vi "Laser Ablation and Capture.vi"() -> ()   [LabVIEW 2016]
uses:
  System.Windows.Forms
  D:/Fabrizio/Labview Projects/VersionControlled/Laser Ablation Capture Software/uc480DotNet.dll
  uc480DotNet.dll
  <vilib>/Utility/miscctls.llb/LVBoundsTypeDef.ctl
  <vilib>/regexp/Match Regular Expression.xnode
  <vilib>/vision/NI_Vision_Development_Module.lvlib
  <vilib>/Utility/config.llb/NI_LVConfig.lvlib
panel:
  in  "Load ROI":bool
  in  "Save current ROI":bool
  in  "Call Last ROI":bool
  in  "Captur time\nConstant":dbl=0.001 min=0.001 step=0.001 format="%#_13g"
  out "Pre-Capture Axis 2":dbl format="%.10e"
  out "Pre-Capture Axis 1":dbl format="%.10e"
  in  "Log files":bool
  out "Axis 2 inverted?":bool
  out "Axis 1 inverted?":bool
  out "Rect height\n(px)":i32
  out "Rect width\n(px)":i32
  in  "Circle?":bool=TRUE
  out "Axis 2 group":i32
  out "Axis 1 group":i32
  in  "Microscope/Capture \nstatus button":bool=TRUE
  in  "X travel":dbl min=0.0 max=150.0 step=0.0001
  in  "Y travel":dbl min=0.0 max=150.0 step=0.0001
  in  "Laser Status":bool
  in  "SINGLE SHOT":bool
  in  "Repetition\nRate (Hz)":dbl=2.34 min=1.0 max=20.0 step=0.01 format="%.2g"
  out "Laser Com Delay":i32
  out "VISA Laser port":string
  in  "Acceleration \n(mm/s²)":dbl=20.0
  out "Camera Status":string="Load parameter"
  in  "Save configuration":bool
  in  "Stages status":bool
  in  "Transparency":u8 max=80 step=1
  in  "Overlay MSI Image":bool
  in  "Home Axes":bool
  out "Axis 2 Offset":dbl
  out "Axis 1 Offset":dbl
  out "Acceleration":dbl
  out "Velocity":dbl
  in  "Axis Initial Parameters":T1={"Velocity (units/seconds)"=1.0, "Acceleration (units/seconds²)"=20.0, "Minimum Jerk Time (seconds)"=0.005, "Maximum Jerk Time (seconds)"=0.009} {"Maximum Jerk Time (seconds)" format="%.6e"; "Minimum Jerk Time (seconds)" format="%.6e"; "Acceleration (units/seconds²)" format="%.6e"; "Velocity (units/seconds)" format="%.6e"}
  out "Axis 2":string
  out "Axis 1":string
  out "XPS_Address":string
  in  "Axes Manual Control":bool
  out "ROI Area \n(mm2)":dbl=4.035870075999999
  out "Laser on/off array":bool[][](array[boolean])
  out "Commands array":string[][](array[string])
  in  "Exit Camera":bool
  in  "Width (px)":i32=240
  in  "X offset":i32=406 step=1
  in  "Y offset":i32=693 step=1
  out "Processi time (sec)":i32=117
  in  "Processing time unit":string(combo)="sec"
  out "Process time":dbl=117.0
  in  "Mode":i32(ring) items=["RGB 32"=0, "RGB 24"=1, "Y8 Monochrom"=6]
  in  "Camera":refnum<k24>(container)
  in  "Init Camera":bool
  in  "Start Live":bool
  in  "Stop Live":bool
  in  "Load Parameter":bool
  out "Error Out":errorcluster caption="error"
  out "Bits/Pixel":i32=32
  out "Width":i32=1280
  out "Height":i32=1024
  out "Serial Number":string="4102944807"
  in  "Camera ID":i32
  in  "Zoom":dbl(ring)=1.5 items=["4X"=4.0, "2X"=2.0, "1.5X"=1.5, "1.25X"=1.25, "1X"=1.0]
  in  "Gain Boost":bool=TRUE
  in  "Snapshot":bool
  out "Output":picture
  in  "Exposure":dbl(slide)=99.80425000000001 min=0.06241666666666667 max=99.80425000000001 step=0.06241666666666667 scale=0.06241666666666667..99.80425000000001 scale format="%#.3g"
  in  "Framerate":dbl(slide)=10.002522802986672 min=0.47411700449083627 max=15.001275108384213 step=0.014032998230481021 scale=0.47411700449083627..15.001275108384213 scale format="%#.3g"
  in  "Pixelclock":i32(slide)=24 min=5 max=40 step=1 scale=5.0..40.0
  in  "error in (no error)":errorcluster
  out "error out":errorcluster
  in  "Precision (%)":dbl=1.0 min=1.0 max=100.0 step=1.0 format="%#_3g"
  in  "Process Image":bool
  in  "Pixel size":dbl=12.19 step=0.01
  in  "Speed (µm/s)":i32=1000
  in  "Heigth (px)":i32=240
  in  "Height \nstep divider":i32=2
  out "Rect height\n(µm/px)":i32=2267
  out "Rect. width \n(µm/px))":i32=2267
  out "Source":T2(plugin-control)
  in  "Open \nManual":bool
  in  "Capture":bool
  out "Log":string
  out "Laser Operation":bool
  in  "LASER":bool
  in  "LAMP":bool
  in  "EXIT":bool
  # "Laser Control"
  # "Stages Control"
  # "Camera Control"
  # "ROI Processing"
  # "Laser spot size and position"
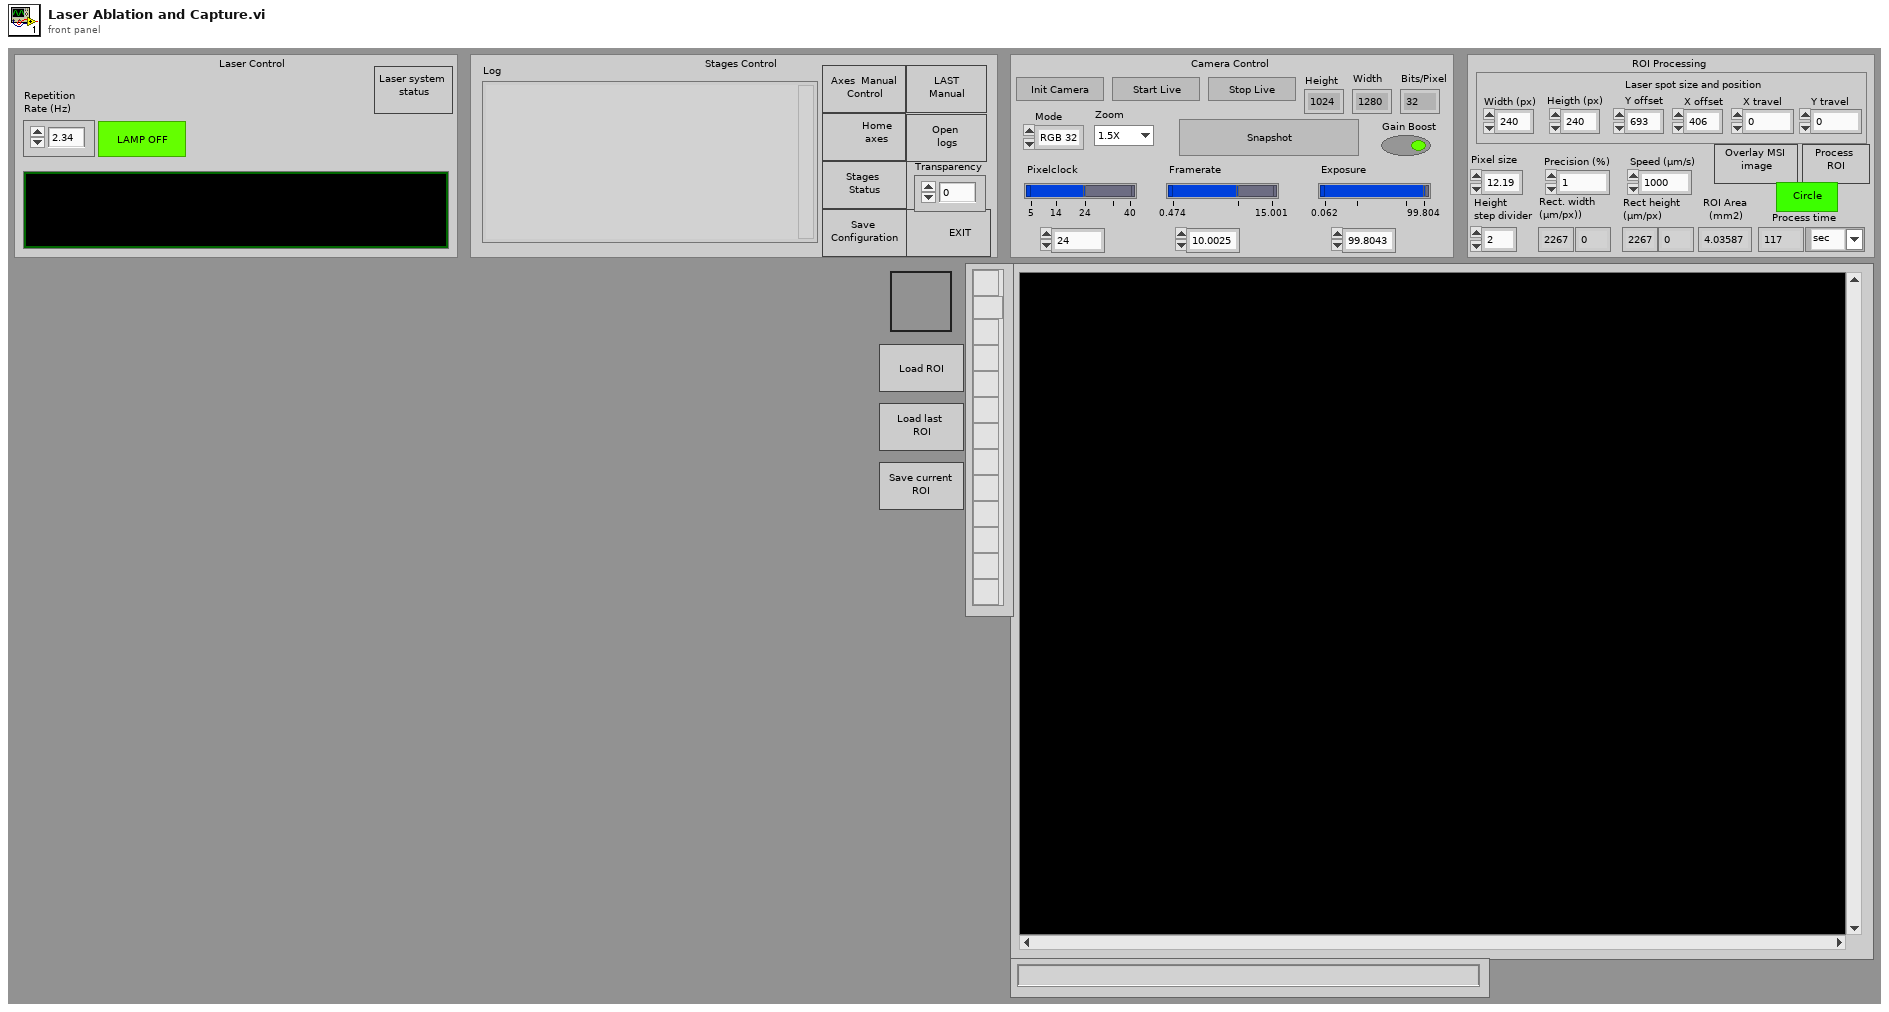
[diagram p1: front panel]
types:
  T1 = cluster{"Velocity (units/seconds)":dbl, "Acceleration (units/seconds²)":dbl, "Minimum Jerk Time (seconds)":dbl, "Maximum Jerk Time (seconds)":dbl}
  T2 = typedef "IMAQ Image.ctl" = refnum<image>
  T3 = typedef "LVBoundsTypeDef.ctl" = cluster{"Width":u32, "Height":u32}
  T4 = enum8{"Enabled", "Disabled", "Disabled and Grayed Out"}
  T5 = typedef "NI_LVConfig.lvlib/Config Data RefNum.ctl" = refnum<k1>
  T6 = enum16{"open", "replace", "create", "open or create", "replace or create", "replace or create with confirmation"}
  T7 = enum32{"Invalid", "Standard", "Closed", "Hidden", "Minimized", "Maximized"}
  T8 = enum32{"invalid app kind", "Development System", "Run Time System", "Student Edition", "Embedded LabVIEW", "Evaluation", "Custom"}
  T9 = cluster{"connection TCP":refnum<k5>, "LogTo File":bool, "Log File refnum":refnum<file>, "no error if error log":bool}
  T10 = cluster{"Global Rectangle":i32[], "Contours":cluster{"Contour Type":u32, "ROI Type":u32, "Points":i32[]}[]}
  T11 = typedef "ROI Descriptor" = cluster{"Global Rectangle":i32[], "Contours":cluster{"ID":enum32{"External", "Internal"}, "Type":u32, "Coordinates":i32[]}[]}
  T12 = cluster{"ID":enum32{"External", "Internal"}, "Type":u32, "Coordinates":i32[]}[]
  T13 = cluster{"ID":enum32{"External", "Internal"}, "Type":u32, "Coordinates":i32[]}
  T14 = cluster{"Contour Type":u32, "ROI Type":u32, "Points":i32[]}[]
  T15 = cluster{"Contour Type":u32, "ROI Type":u32, "Points":i32[]}
diagram:
  w63 = 682  # Height
  w64 = 853  # Width
  w65 = 1 items=["None", "FixedSingle", "Fixed3D"]  # BorderStyle
  w69 = u8 2  # Deaktiviert
  w70 = u8 2  # Deaktiviert
  w72 = u8 2  # Deaktiviert
  w73 = u8 0  # Deaktiviert
  # "Button and controls"
  # "Camera control buttons"
  n1 = property on="Property Node" class="PictureBox"(reference="Camera", "BorderStyle"=w65, "Width"=w64, "Height"=w63) -> (reference out=w53:refnum<k24>, error out=w54:errorcluster)  [unwired: 1 in]
  n2 = property on="Property Node" class="PictureBox"(reference=w53, error in=w54) -> (reference out=w52:refnum<k24>, error out=w51:errorcluster, "Handle"=w50:refnum<k24>)
  n3 = while "Camera Control" {
    shift-right: [w82] -> _
    shift-left: w51 -> [w88]
    shift-right: [w85] -> _
    shift-left: _ -> [w78]
    shift-right: [w80] -> _
    shift-left: w52 -> [w81]
    tunnel: w50 -> [w79]
    stop <- w86 stop-if-true
    # ".NetReference"
    # ".Net Reference"
    n4 = event shown="[1] Timeout" {
      selector: _ -> [_ _]
      dyn-events: _ -> [_ _]
      timeout: 0 -> [_ _]
      event "Load Parameter", "Start Live": Mouse Down {
        n5 = event-data() -> ()  [unwired: 1 in, 2 out]
      }
      event Timeout {
        n6 = event-data() -> ()  [unwired: 1 in, 2 out]
      }
    }
    n7 = event shown="[1] Timeout" {
      selector: _ -> [_ _]
      dyn-events: _ -> [_ _]
      timeout: 0 -> [_ _]
      tunnel: [w102 w113] -> w89
      tunnel: w88 -> [w112 w113]
      tunnel: w78 -> [w111 _]
      event "Pixelclock": Value Change; "Pixelclock": Mouse Move; "Pixelclock": Key Down; "Pixelclock": Mouse Up {
        n8 = event-data() -> ("CtlRef"=w104:refnum<vi>)  [unwired: 1 in, 3 out]
        n9 = call "uc480_SubVI_Example_GetFramerate.vi"(".NET (Reference)"=w111, "Error In"=w112) -> ("Framerate"=w110:dbl, "Inc"=w109:dbl, "Min"=w107:dbl, "Max"=w108:dbl, "error out"=w106:errorcluster)  [unwired: 9 in]
        n10 = property on="Framerate" class="Slide (strict)"(error in=w106, "Value"=w110, "Increment"=w109, "Minimum"=w107, "Maximum"=w108) -> (error out=w105:errorcluster)  [unwired: 1 in, 1 out]
        n11 = property on="Framerate" class="Slide (strict)"(error in=w105, "Scale.Increment"=w109, "Scale.Minimum"=w107, "Scale.Maximum"=w108) -> (error out=w103:errorcluster)  [unwired: 1 in, 1 out]
        n12 = Close Reference(reference=w104, error in (no error)=w103) -> (error out=w102:errorcluster)
      }
      event Timeout {
        n13 = event-data() -> ()  [unwired: 1 in, 2 out]
      }
    }
    n14 = case shown="False" "Load Parameter" {
      tunnel: ["" "Load parameter"] -> w95
      frame False {
      }
      frame True {
      }
    }
    n15 = case shown="False" "Init Camera" {
      tunnel: ["" "Init camera"] -> w99
      frame False {
      }
      frame True {
      }
    }
    n16 = case shown="False" "Exit Camera" {
      tunnel: ["" "Exit camera"] -> w93
      frame False {
      }
      frame True {
      }
    }
    n17 = event shown="[1] Timeout" {
      selector: _ -> [_ _]
      dyn-events: _ -> [_ _]
      timeout: 0 -> [_ _]
      tunnel: w89 -> [w124 w125]
      tunnel: [w114 w125] -> w91
      tunnel: w78 -> [w123 _]
      event "Pixelclock", "Framerate": Value Change; "Pixelclock", "Framerate": Mouse Move; "Pixelclock", "Framerate": Key Down; "Pixelclock", "Framerate": Mouse Up {
        n18 = event-data() -> ("CtlRef"=w116:refnum<vi>)  [unwired: 1 in, 3 out]
        n19 = call "uc480_SubVI_Example_GetExposure.vi"(".NET (Reference)"=w123, "Error In"=w124) -> ("Exposure"=w120:dbl, "Inc"=w119:dbl, "Min"=w118:dbl, "Max"=w117:dbl, "Error out"=w121:errorcluster)  [unwired: 9 in]
        n20 = property on="Exposure" class="Slide (strict)"(error in=w121, "Value"=w120, "Increment"=w119, "Minimum"=w118, "Maximum"=w117) -> (error out=w122:errorcluster)  [unwired: 1 in, 1 out]
        n21 = property on="Exposure" class="Slide (strict)"(error in=w122, "Scale.Increment"=w119, "Scale.Minimum"=w118, "Scale.Maximum"=w117) -> (error out=w115:errorcluster)  [unwired: 1 in, 1 out]
        n22 = Close Reference(reference=w116, error in (no error)=w115) -> (error out=w114:errorcluster)
      }
      event Timeout {
        n23 = event-data() -> ()  [unwired: 1 in, 2 out]
      }
    }
    n24 = case shown="False" "Start Live" {
      tunnel: ["" "Start live"] -> w98
      frame False {
      }
      frame True {
      }
    }
    n25 = case shown="False" "Stop Live" {
      tunnel: ["" "Stop live"] -> w94
      frame False {
      }
      frame True {
      }
    }
    n26 = local read "Camera Status"() -> (w75:string)
    n27 = Concatenate Strings(w99, w98, w95, w94, w93) -> (→"Camera Status":string)
    n28 = case shown="Default" w75 {
      tunnel: w78 -> [w168 w208 w266 w308 w488 w547]
      tunnel: w91 -> [w171 w209 w267 w318 w487 w548]
      tunnel: [w142 w207 w275 w317 w446 w546] -> w85
      tunnel: [w143 w206 w276 w316 w483 w544] -> w84
      tunnel: [FALSE FALSE TRUE FALSE FALSE FALSE] -> w86
      tunnel: w81 -> [w141 w200 w248 w300 w441 w537]
      tunnel: [w141 w200 w247 w299 w441 w537] -> w80
      tunnel: w79 -> [_ _ _ w296 _ _]
      frame "Load parameter" {
        # "SubVI Example for \nMemory allocation"
        # "Is acquisition running?"
        # "Load Parameter"
        n29 = property class="Camera"(reference=w168, error in=w171) -> (error out=w176:errorcluster, "Acquisition"=w175:refnum<k24>)  [unwired: 1 out]
        n30 = invoke class="Acquisition" method="HasStarted"(reference=w175, error in=w176) -> (reference out=w172:refnum<k24>, error out=w174:errorcluster, "bValue"=w170:bool)  [unwired: 2 in, 1 out]
        n31 = control-ref of="Start Live"() -> (w166:refnum<vi>)
        n32 = invoke class="Acquisition" method="ToString"(reference=w172, error in=w174) -> (reference out=w138:refnum<k24>, error out=w137:errorcluster, "ToString"=w173:string)  [unwired: 1 in]
        n33 = property class="Bool"(reference=w166, "Disabled"=u8 0 ("Deaktiviert")) -> (reference out=w140:refnum<vi>, error out=w139:errorcluster)  [unwired: 1 in]
        n34 = Close Reference(reference=w138, error in (no error)=w137) -> (error out=w136:errorcluster)
        n35 = Close Reference(reference=w140, error in (no error)=w139) -> ()  [unwired: 1 out]
        n36 = call "uc480_Error_Handling.vi"("Error String"=w173, "Error In"=w136) -> ("Error Out"=w169:errorcluster)  [unwired: 9 in]
        n37 = case shown="False" w170 {
          tunnel: w169 -> [w184 w191]
          tunnel: w168 -> [w182 w192]
          tunnel: [w183 w191] -> w167
          tunnel: [w182 w192] -> w142
          frame False {
            n38 = property class="Camera"(reference=w182, error in=w184) -> (error out=w186:errorcluster, "Parameter"=w185:refnum<k24>)  [unwired: 1 out]
            n39 = invoke class="Parameter" method="Load"(reference=w185, error in=w186, "strFilename"="") -> (reference out=w188:refnum<k24>, error out=w189:errorcluster, "Load"=w181:i32)  [unwired: 1 in, 1 out]
            n40 = invoke class="Parameter" method="ToString"(reference=w188, error in=w189) -> (reference out=w178:refnum<k24>, error out=w180:errorcluster, "ToString"=w190:string)  [unwired: 1 in]
            n41 = Close Reference(reference=w178, error in (no error)=w180) -> (error out=w179:errorcluster)
            n42 = call "uc480_Error_Handling.vi"("Error Code"=w181, "Error String"=w190, "Error In"=w179) -> ("Error Out"=w183:errorcluster)  [unwired: 8 in]
          }
          frame True {
          }
        }
        n43 = call "uc480_SubVI_Example_MemoryAllocation.vi"(".NET (Reference)"=w142, "Error In"=w167) -> ("Error Out"=w144:errorcluster)  [unwired: 13 in, 4 out]
        n44 = call "uc480_SubVI_Example_GetPixelClock.vi"(".NET (Reference)"=w142, "Error In"=w144) -> ("Pixel Clock"=w145:i32, "Inc"=w147:i32, "Min"=w148:i32, "Max"=w149:i32, "error out"=w146:errorcluster)  [unwired: 9 in]
        n45 = property on="Pixelclock" class="Slide (strict)"(error in=w146, "Value"=w145, "Increment"=w147, "Minimum"=w148, "Maximum"=w149) -> (error out=w150:errorcluster)  [unwired: 1 in, 1 out]
        n46 = property on="Pixelclock" class="Slide (strict)"(error in=w150, "Scale.Increment"=w147, "Scale.Minimum"=w148, "Scale.Maximum"=w149) -> (error out=w151:errorcluster)  [unwired: 1 in, 1 out]
        n47 = call "uc480_SubVI_Example_GetFramerate.vi"(".NET (Reference)"=w142, "Error In"=w151) -> ("Framerate"=w154:dbl, "Inc"=w155:dbl, "Min"=w156:dbl, "Max"=w157:dbl, "error out"=w153:errorcluster)  [unwired: 9 in]
        n48 = property on="Framerate" class="Slide (strict)"(error in=w153, "Value"=w154, "Increment"=w155, "Minimum"=w156, "Maximum"=w157) -> (error out=w152:errorcluster)  [unwired: 1 in, 1 out]
        n49 = property on="Framerate" class="Slide (strict)"(error in=w152, "Scale.Increment"=w155, "Scale.Minimum"=w156, "Scale.Maximum"=w157) -> (error out=w158:errorcluster)  [unwired: 1 in, 1 out]
        n50 = call "uc480_SubVI_Example_GetExposure.vi"(".NET (Reference)"=w142, "Error In"=w158) -> ("Exposure"=w161:dbl, "Inc"=w162:dbl, "Min"=w163:dbl, "Max"=w164:dbl, "Error out"=w159:errorcluster)  [unwired: 9 in]
        n51 = property on="Exposure" class="Slide (strict)"(error in=w159, "Value"=w161, "Increment"=w162, "Minimum"=w163, "Maximum"=w164) -> (error out=w160:errorcluster)  [unwired: 1 in, 1 out]
        n52 = property on="Exposure" class="Slide (strict)"(error in=w160, "Scale.Increment"=w162, "Scale.Minimum"=w163, "Scale.Maximum"=w164) -> (error out=w143:errorcluster)  [unwired: 1 in, 1 out]
      }
      frame "Stop live" {
        # "Is acquisition running?"
        # "Stop Acquisition"
        n53 = property class="Camera"(reference=w208, error in=w209) -> (error out=w216:errorcluster, "Acquisition"=w215:refnum<k24>)  [unwired: 1 out]
        n54 = invoke class="Acquisition" method="HasStarted"(reference=w215, error in=w216) -> (reference out=w210:refnum<k24>, error out=w212:errorcluster, "bValue"=w214:bool)  [unwired: 2 in, 1 out]
        n55 = control-ref of="Load Parameter"() -> (w204:refnum<vi>)
        n56 = control-ref of="Start Live"() -> (w201:refnum<vi>)
        n57 = invoke class="Acquisition" method="ToString"(reference=w210, error in=w212) -> (reference out=w193:refnum<k24>, error out=w195:errorcluster, "ToString"=w211:string)  [unwired: 1 in]
        n58 = property class="Bool"(reference=w204, "Disabled"=u8 0 ("Deaktiviert")) -> (reference out=w199:refnum<vi>, error out=w198:errorcluster)  [unwired: 1 in]
        n59 = property class="Bool"(reference=w201, "Disabled"=u8 0 ("Deaktiviert")) -> (reference out=w197:refnum<vi>, error out=w196:errorcluster)  [unwired: 1 in]
        n60 = Close Reference(reference=w193, error in (no error)=w195) -> (error out=w194:errorcluster)
        n61 = Close Reference(reference=w199, error in (no error)=w198) -> ()  [unwired: 1 out]
        n62 = Close Reference(reference=w197, error in (no error)=w196) -> ()  [unwired: 1 out]
        n63 = call "uc480_Error_Handling.vi"("Error String"=w211, "Error In"=w194) -> ("Error Out"=w213:errorcluster)  [unwired: 9 in]
        n64 = case shown="True" w214 {
          tunnel: [w218 w237] -> w206
          tunnel: w213 -> [w218 w238]
          tunnel: w208 -> [w217 w230]
          tunnel: [w217 w230] -> w207
          frame False {
          }
          frame True {
            n65 = property class="Camera"(reference=w230, error in=w238) -> (error out=w234:errorcluster, "Acquisition"=w235:refnum<k24>)  [unwired: 1 out]
            n66 = invoke class="Acquisition" method="Stop"(reference=w235, error in=w234) -> (reference out=w232:refnum<k24>, error out=w233:errorcluster, "Stop"=w231:i32)  [unwired: 1 in]
            n67 = invoke class="Acquisition" method="ToString"(reference=w232, error in=w233) -> (reference out=w227:refnum<k24>, error out=w229:errorcluster, "ToString"=w236:string)  [unwired: 1 in]
            n68 = Close Reference(reference=w227, error in (no error)=w229) -> (error out=w228:errorcluster)
            n69 = call "uc480_Error_Handling.vi"("Error Code"=w231, "Error String"=w236, "Error In"=w228) -> ("Error Out"=w237:errorcluster)  [unwired: 8 in]
            n70 = Get Date/Time In Seconds() -> (seconds since 1Jan1904=w225:timestamp)
            n71 = Format Date/Time String(time format string (%c)="%m/%d/%y - %I:%M %p  ", seconds (now)=w225) -> (date/time string=w226:string)  [unwired: 1 in]
            n72 = Concatenate Strings(w226, "Camera stopped", "\r") -> (w221:string)
            n73 = invoke on="Log" class="Str" method="Append String"("string"=w221) -> (error out=w219:errorcluster)  [unwired: 3 in, 3 out]
            n74 = property on="Log" class="Str"(error in=w219, "Text.Scroll Position"=u32 500000) -> ()  [unwired: 1 in, 2 out]
          }
        }
      }
      frame "Exit camera" {
        # "Close .Net Reference"
        # "Is acquisition running?"
        # "Stop Acquisition"
        # "Close Camera"
        n75 = property class="Camera"(reference=w266, error in=w267) -> (error out=w274:errorcluster, "Acquisition"=w273:refnum<k24>)  [unwired: 1 out]
        n76 = invoke class="Acquisition" method="HasStarted"(reference=w273, error in=w274) -> (reference out=w268:refnum<k24>, error out=w270:errorcluster, "bValue"=w272:bool)  [unwired: 2 in, 1 out]
        n77 = control-ref of="Load Parameter"() -> (w257:refnum<vi>)
        n78 = control-ref of="Init Camera"() -> (w259:refnum<vi>)
        n79 = control-ref of="Start Live"() -> (w258:refnum<vi>)
        n80 = control-ref of="Stop Live"() -> (w256:refnum<vi>)
        n81 = invoke class="Acquisition" method="ToString"(reference=w268, error in=w270) -> (reference out=w253:refnum<k24>, error out=w255:errorcluster, "ToString"=w269:string)  [unwired: 1 in]
        n82 = property class="Bool"(reference=w258, "Disabled"=u8 0 ("Deaktiviert")) -> (reference out=w242:refnum<vi>, error out=w241:errorcluster)  [unwired: 1 in]
        n83 = property class="Bool"(reference=w259, "Disabled"=u8 0 ("Deaktiviert")) -> (reference out=w240:refnum<vi>, error out=w239:errorcluster)  [unwired: 1 in]
        n84 = property class="Bool"(reference=w257, "Disabled"=u8 0 ("Deaktiviert")) -> (reference out=w244:refnum<vi>, error out=w243:errorcluster)  [unwired: 1 in]
        n85 = property class="Bool"(reference=w256, "Disabled"=u8 0 ("Deaktiviert")) -> (reference out=w246:refnum<vi>, error out=w245:errorcluster)  [unwired: 1 in]
        n86 = Close Reference ("Close Referenz")(reference=w253, error in (no error)=w255) -> (error out=w254:errorcluster)
        n87 = Close Reference(reference=w242, error in (no error)=w241) -> ()  [unwired: 1 out]
        n88 = Close Reference(reference=w240, error in (no error)=w239) -> ()  [unwired: 1 out]
        n89 = Close Reference(reference=w246, error in (no error)=w245) -> ()  [unwired: 1 out]
        n90 = Close Reference(reference=w244, error in (no error)=w243) -> ()  [unwired: 1 out]
        n91 = call "uc480_Error_Handling.vi"("Error String"=w269, "Error In"=w254) -> ("Error Out"=w271:errorcluster)  [unwired: 9 in]
        n92 = case shown="True" w272 {
          tunnel: [w283 w294] -> w264
          tunnel: w271 -> [w283 w295]
          tunnel: w266 -> [w282 w287]
          tunnel: [w282 w287] -> w265
          frame False {
          }
          frame True {
            n93 = property class="Camera"(reference=w287, error in=w295) -> (error out=w291:errorcluster, "Acquisition"=w292:refnum<k24>)  [unwired: 1 out]
            n94 = invoke class="Acquisition" method="Stop"(reference=w292, error in=w291) -> (reference out=w289:refnum<k24>, error out=w290:errorcluster, "Stop"=w288:i32)  [unwired: 1 in]
            n95 = invoke class="Acquisition" method="ToString"(reference=w289, error in=w290) -> (reference out=w284:refnum<k24>, error out=w286:errorcluster, "ToString"=w293:string)  [unwired: 1 in]
            n96 = Close Reference ("Close Referenz")(reference=w284, error in (no error)=w286) -> (error out=w285:errorcluster)
            n97 = call "uc480_Error_Handling.vi"("Error Code"=w288, "Error String"=w293, "Error In"=w285) -> ("Error Out"=w294:errorcluster)  [unwired: 8 in]
          }
        }
        n98 = invoke class="Camera" method="Exit"(reference=w265, error in=w264) -> (reference out=w275:refnum<k24>, error out=w278:errorcluster, "Exit"=w277:i32)  [unwired: 1 in]
        n99 = invoke class="Camera" method="ToString"(reference=w275, error in=w278) -> (error out=w279:errorcluster, "ToString"=w280:string)  [unwired: 1 in, 1 out]
        n100 = call "uc480_Error_Handling.vi"("Error Code"=w277, "Error String"=w280, "Error In"=w279) -> ("Error Out"=w252:errorcluster)  [unwired: 8 in]
        n101 = property class="PictureBox"(reference=w248, error in=w252, "Width"=853, "Height"=682) -> (reference out=w247:refnum<k24>, error out=w251:errorcluster)
        n102 = Close Reference ("Close Referenz")(reference=w275, error in (no error)=w251) -> (error out=w276:errorcluster)
      }
      frame Default {
        # "SubVI Example for Timing"
        # "Has acquisition started?"
        n103 = call "uc480_SubVI_Example_Timing.vi"(".NET (Reference)"=w308, "Pixelclock"="Pixelclock", "Exposure time"="Exposure", "Framerate"="Framerate", "Error In"=w318) -> ("Pixelclock"=w311:i32, "Exposure time"=w310:dbl, "Framerate"=w309:dbl, "Error Out"=w315:errorcluster)  [unwired: 7 in]
        n104 = property on="Framerate" class="Schieber (strikt)"(error in=w315, "Scale.RngStart"=w309) -> (error out=w314:errorcluster)  [unwired: 1 in, 1 out]
        n105 = property on="Exposure" class="Schieber (strikt)"(error in=w314, "Scale.RngStart"=w310) -> (error out=w313:errorcluster)  [unwired: 1 in, 1 out]
        n106 = property on="Pixelclock" class="Schieber (strikt)"(error in=w313, "Scale.RngStart"=w311) -> (error out=w312:errorcluster)  [unwired: 1 in, 1 out]
        n107 = property class="Camera"(reference=w308, error in=w312) -> (reference out=w301:refnum<k24>, error out=w324:errorcluster, "Acquisition"=w323:refnum<k24>)
        n108 = invoke class="Acquisition" method="HasStarted"(reference=w323, error in=w324) -> (reference out=w298:refnum<k24>, error out=w320:errorcluster, "HasStarted"=w319:i32, "bValue"=w297:bool)  [unwired: 2 in]
        n109 = invoke class="Acquisition" method="ToString"(reference=w298, error in=w320) -> (reference out=w302:refnum<k24>, error out=w322:errorcluster, "ToString"=w321:string)  [unwired: 1 in]
        n110 = call "uc480_Error_Handling.vi"("Error Code"=w319, "Error String"=w321, "Error In"=w322) -> ("Error Out"=w304:errorcluster)  [unwired: 8 in]
        n111 = Close Reference(reference=w302, error in (no error)=w304) -> (error out=w303:errorcluster)
        n112 = case "Show Image" shown="True" w297 {
          tunnel: [w328 w340] -> w316
          tunnel: w303 -> [w328 w368]
          tunnel: w301 -> [w327 w332]
          tunnel: [w327 w336] -> w317
          tunnel: w300 -> [w326 w357]
          tunnel: [w326 w334] -> w299
          tunnel: w296 -> [_ w364]
          frame False {
            (unwired) ""
          }
          frame True {
            n113 = local read "Height"() -> (w361:i32)
            n114 = local read "Width"() -> (w362:i32)
            n115 = Quotient & Remainder(x=w362, y="Zoom") -> (floor(x/y)=w359:dbl)  [unwired: 1 out]
            n116 = Quotient & Remainder(x=w361, y="Zoom") -> (floor(x/y)=w358:dbl)  [unwired: 1 out]
            n117 = To Long Integer(number=w359) -> (32bit integer=w331:i32)
            n118 = To Long Integer(number=w358) -> (32bit integer=w330:i32)
            n119 = property class="PictureBox"(reference=w357, error in=w368, "Width"=w331, "Height"=w330) -> (reference out=w334:refnum<k24>, error out=w363:errorcluster)
            n120 = property class="Camera"(reference=w332, error in=w363) -> (reference out=w333:refnum<k24>, error out=w370:errorcluster, "Memory"=w371:refnum<k24>)
            n121 = invoke class="Memory" method="GetActive"(reference=w371, error in=w370) -> (reference out=w365:refnum<k24>, error out=w366:errorcluster, "s32MemId"=w337:i32)  [unwired: 2 in, 1 out]
            n122 = property class="Camera"(reference=w333, error in=w366) -> (reference out=w345:refnum<k24>, error out=w369:errorcluster, "Display"=w354:refnum<k24>)
            n123 = invoke class="Display" method="Render"(reference=w354, error in=w369, "memID"=w337, "windowHandle"=w364) -> (reference out=w355:refnum<k24>, error out=w356:errorcluster)  [unwired: 1 in, 3 out]
            n124 = property class="Camera"(reference=w345, error in=w356) -> (reference out=w336:refnum<k24>, error out=w352:errorcluster, "Gain"=w350:refnum<k24>)
            n125 = property class="Gain"(reference=w350, error in=w352) -> (reference out=w351:refnum<k24>, error out=w347:errorcluster, "Hardware"=w346:refnum<k24>)
            n126 = property class="GainHardware"(reference=w346, error in=w347) -> (reference out=w343:refnum<k24>, error out=w348:errorcluster, "Boost"=w349:refnum<k24>)
            n127 = property class="GainBoost"(reference=w349, error in=w348, "Enabled"="Gain Boost") -> (reference out=w344:refnum<k24>, error out=w335:errorcluster)
            n128 = case "Snapshot control" shown="True" "Snapshot" {
              tunnel: w332 -> [_ w392]
              tunnel: w335 -> [w372 w396]
              tunnel: [w372 w383] -> w329
              tunnel: w331 -> [_ w386]
              tunnel: w330 -> [_ w385]
              frame False {
              }
              frame True {
                n129 = property class="Camera"(reference=w392, error in=w396) -> (error out=w416:errorcluster, "Memory"=w415:refnum<k24>)  [unwired: 1 out]
                n130 = local read "Zoom"() -> (w391:dbl)
                n131 = invoke class="Memory" method="GetList"(reference=w415, error in=w416) -> (reference out=w421:refnum<k24>, error out=w420:errorcluster, "GetList"=w422:i32, "idList"=w409:i32[])  [unwired: 2 in]
                n132 = Bundle(cluster=T3 {"Width"=0, "Height"=0} ("Draw Area Size"), "Width"=w386, "Height"=w385) -> (w387:T3)
                n133 = Divide(x=1.0, y=w391) -> (x/y=w389:dbl)
                n134 = property on="Output" class="Pict"("ZoomFactor"=w389, "Draw Area Size"=w387) -> ()  [unwired: 2 in, 2 out]
                n135 = invoke class="Memory" method="ToString"(reference=w421, error in=w420) -> (reference out=w394:refnum<k24>, error out=w404:errorcluster, "ToString"=w419:string)  [unwired: 1 in]
                n136 = Index Array(array=w409, index=0 ("Active \nAcquisition Buffer")) -> (element=w406:i32)
                n137 = Index Array(array=w409, index=u32 0 ("Active \nOutput Buffer")) -> (element=w405:i32)
                n138 = Close Reference(reference=w394, error in (no error)=w404) -> (error out=w403:errorcluster)
                n139 = call "uc480_Error_Handling.vi"("Error Code"=w422, "Error String"=w419, "Error In"=w403) -> ("Error Out"=w412:errorcluster)  [unwired: 8 in]
                n140 = Get Date/Time In Seconds() -> (seconds since 1Jan1904=w376:timestamp)
                n141 = property class="Camera"(reference=w392, error in=w412) -> (error out=w411:errorcluster, "Memory"=w410:refnum<k24>)  [unwired: 1 out]
                n142 = Format Date/Time String(time format string (%c)="%m/%d/%y -%I:%M %p  ", seconds (now)=w376) -> (date/time string=w375:string)  [unwired: 1 in]
                n143 = invoke class="Memory" method="SetActive"(reference=w410, error in=w411, "s32MemId"=w406) -> (reference out=w395:refnum<k24>, error out=w402:errorcluster)  [unwired: 1 in, 2 out]
                n144 = Concatenate Strings(w375, "Snapshot taken", "\r") -> (w380:string)
                n145 = Close Reference(reference=w395, error in (no error)=w402) -> (error out=w401:errorcluster)
                n146 = invoke on="Log" class="Str" method="Append String"("string"=w380) -> (error out=w373:errorcluster)  [unwired: 3 in, 3 out]
                n147 = property class="Camera"(reference=w392, error in=w401) -> (error out=w418:errorcluster, "Memory"=w407:refnum<k24>)  [unwired: 1 out]
                n148 = invoke class="Memory" method="CopyToArray"(reference=w407, error in=w418, "s32MemId"=w405) -> (reference out=w397:refnum<k24>, error out=w398:errorcluster, "u8Image"=w417:u8[])  [unwired: 2 in, 2 out]
                n149 = property on="Log" class="Str"(error in=w373, "Text.Scroll Position"=u32 500000) -> ()  [unwired: 1 in, 2 out]
                n150 = invoke class="Memory" method="ToString"(reference=w397, error in=w398) -> (reference out=w393:refnum<k24>, error out=w400:errorcluster, "ToString"=w423:string)  [unwired: 1 in]
                n151 = Close Reference(reference=w393, error in (no error)=w400) -> (error out=w399:errorcluster)
                n152 = call "uc480_Error_Handling.vi"("Error String"=w423, "Error In"=w399) -> ("Error Out"=w414:errorcluster)  [unwired: 9 in]
                n153 = call "uc480_ArrayToImage.vi"("Error In"=w414, "InArray"=w417, ".NET (Reference)"=w392) -> ("Error Out"=w382:errorcluster, "Image"=w384:picture)  [unwired: 7 in]
                "Output" <- w384
                n154 = call "Picture to IMAQ.vi"("Error In"=w382, "picture"=w384) -> ("Error Out"=w383:errorcluster, "Image"=→"Source":T2)  [unwired: 8 in]
              }
            }
            n155 = Close Reference(reference=w343, error in (no error)=w329) -> (error out=w342:errorcluster)
            n156 = Close Reference(reference=w344, error in (no error)=w342) -> (error out=w339:errorcluster)
            n157 = Close Reference(reference=w351, error in (no error)=w339) -> (error out=w353:errorcluster)
            n158 = Close Reference(reference=w355, error in (no error)=w353) -> (error out=w367:errorcluster)
            n159 = Close Reference(reference=w365, error in (no error)=w367) -> (error out=w340:errorcluster)
          }
        }
      }
      frame "Init camera" {
        # "SubVI Example for \nGetDefault Timing"
        # "SubVI Example for \nMemory allocation"
        # "SubVI Example for \nTiming"
        # "SubVI Example for \nCamera Init"
        # "Pixelformat"
        n160 = control-ref of="Load Parameter"() -> (w447:refnum<vi>)
        n161 = call "uc480_SubVI_Example_CameraInit.vi"("Error In"=w487, "Camera ID"="Camera ID", "Init Camera Flag"=TRUE, ".NET (Reference)"=w488) -> ("Error Out"=w493:errorcluster, ".NET (Reference)"=w446:refnum<k24>)  [unwired: 6 in]
        n162 = control-ref of="Init Camera"() -> (w451:refnum<vi>)
        n163 = control-ref of="Start Live"() -> (w449:refnum<vi>)
        n164 = property on="Property Node" class="Camera"(reference=w446, error in=w493) -> (error out=w494:errorcluster, "PixelFormat"=w495:refnum<k24>)  [unwired: 1 out]
        n165 = property class="Bool"(reference=w449, "Disabled"=u8 0 ("Deaktiviert")) -> (reference out=w438:refnum<vi>, error out=w437:errorcluster)  [unwired: 1 in]
        n166 = property class="Bool"(reference=w451, "Disabled"=u8 2 ("Deaktiviert")) -> (reference out=w440:refnum<vi>, error out=w439:errorcluster)  [unwired: 1 in]
        n167 = property class="Bool"(reference=w447, "Disabled"=u8 0 ("Deaktiviert")) -> (reference out=w436:refnum<vi>, error out=w435:errorcluster)  [unwired: 1 in]
        n168 = Close Reference(reference=w438, error in (no error)=w437) -> ()  [unwired: 1 out]
        n169 = Close Reference(reference=w440, error in (no error)=w439) -> ()  [unwired: 1 out]
        n170 = Close Reference(reference=w436, error in (no error)=w435) -> ()  [unwired: 1 out]
        n171 = invoke class="PixelFormat" method="Set"(reference=w495, error in=w494, "mode"="Mode") -> (reference out=w491:refnum<k24>, error out=w484:errorcluster, "Set"=w490:i32)  [unwired: 1 in, 1 out]
        n172 = Get Date/Time In Seconds() -> (seconds since 1Jan1904=w427:timestamp)
        n173 = Format Date/Time String(time format string (%c)="%m/%d/%y - %I:%M %p  ", seconds (now)=w427) -> (date/time string=w426:string)  [unwired: 1 in]
        n174 = invoke class="PixelFormat" method="ToString"(reference=w491, error in=w484) -> (reference out=w432:refnum<k24>, error out=w434:errorcluster, "ToString"=w492:string)  [unwired: 1 in]
        n175 = Concatenate Strings(w426, "Camera Initialized", "\r") -> (w431:string)
        n176 = Close Reference(reference=w432, error in (no error)=w434) -> (error out=w433:errorcluster)
        n177 = call "uc480_Error_Handling.vi"("Error Code"=w490, "Error String"=w492, "Error In"=w433) -> ("Error Out"=w458:errorcluster)  [unwired: 8 in]
        n178 = invoke on="Log" class="Str" method="Append String"("string"=w431) -> (error out=w424:errorcluster)  [unwired: 3 in, 3 out]
        n179 = property on="Log" class="Str"(error in=w424, "Text.Scroll Position"=u32 500000) -> ()  [unwired: 1 in, 2 out]
        n180 = call "uc480_SubVI_Example_GetDefault_Timing.vi"(".NET (Reference)"=w446, "Error In"=w458) -> ("Pixelclock"=w457:i32, "Exposure time"=w456:dbl, "Framerate"=w455:dbl, "Error Out"=w454:errorcluster)  [unwired: 10 in]
        n181 = call "uc480_SubVI_Example_GetPixelClock.vi"(".NET (Reference)"=w446, "Error In"=w454) -> ("Pixel Clock"=w459:i32, "Inc"=w461:i32, "Min"=w462:i32, "Max"=w463:i32, "error out"=w460:errorcluster)  [unwired: 9 in]
        n182 = property on="Pixelclock" class="Slide (strict)"(error in=w460, "Value"=w459, "Increment"=w461, "Minimum"=w462, "Maximum"=w463) -> (error out=w464:errorcluster)  [unwired: 1 in, 1 out]
        n183 = property on="Pixelclock" class="Slide (strict)"(error in=w464, "Scale.Increment"=w461, "Scale.Minimum"=w462, "Scale.Maximum"=w463) -> (error out=w465:errorcluster)  [unwired: 1 in, 1 out]
        n184 = call "uc480_SubVI_Example_GetFramerate.vi"(".NET (Reference)"=w446, "Error In"=w465) -> ("Framerate"=w468:dbl, "Inc"=w469:dbl, "Min"=w470:dbl, "Max"=w471:dbl, "error out"=w467:errorcluster)  [unwired: 9 in]
        n185 = property on="Framerate" class="Slide (strict)"(error in=w467, "Value"=w468, "Increment"=w469, "Minimum"=w470, "Maximum"=w471) -> (error out=w466:errorcluster)  [unwired: 1 in, 1 out]
        n186 = property on="Framerate" class="Slide (strict)"(error in=w466, "Scale.Increment"=w469, "Scale.Minimum"=w470, "Scale.Maximum"=w471) -> (error out=w472:errorcluster)  [unwired: 1 in, 1 out]
        n187 = call "uc480_SubVI_Example_GetExposure.vi"(".NET (Reference)"=w446, "Error In"=w472) -> ("Exposure"=w475:dbl, "Inc"=w476:dbl, "Min"=w477:dbl, "Max"=w478:dbl, "Error out"=w473:errorcluster)  [unwired: 9 in]
        n188 = property on="Exposure" class="Slide (strict)"(error in=w473, "Value"=w475, "Increment"=w476, "Minimum"=w477, "Maximum"=w478) -> (error out=w474:errorcluster)  [unwired: 1 in, 1 out]
        n189 = property on="Exposure" class="Slide (strict)"(error in=w474, "Scale.Increment"=w476, "Scale.Minimum"=w477, "Scale.Maximum"=w478) -> (error out=w453:errorcluster)  [unwired: 1 in, 1 out]
        n190 = call "uc480_SubVI_Example_Timing.vi"(".NET (Reference)"=w446, "Pixelclock"=w457, "Exposure time"=w456, "Framerate"=w455, "Error In"=w453) -> ("Error Out"=w445:errorcluster)  [unwired: 7 in, 3 out]
        n191 = call "uc480_SubVI_Example_Is_XS.vi"("Error In"=w445, ".NET (Reference)"=w446) -> ("Error Out"=w442:errorcluster, "IsXS"=w444:bool)  [unwired: 7 in, 1 out]
        n192 = case shown="False" w444 {
          tunnel: w442 -> [w509 w522]
          tunnel: [w509 w522] -> w443
          frame False {
            n193 = control-ref of="Pixelclock"() -> (w505:refnum<vi>)
            n194 = control-ref of="Framerate"() -> (w504:refnum<vi>)
            n195 = control-ref of="Exposure"() -> (w503:refnum<vi>)
            n196 = property class="Slide (strict)"(reference=w505, "DisabledEnum"=T4."Enabled" ("Disabled")) -> (reference out=w502:refnum<vi>, error out=w501:errorcluster)  [unwired: 1 in]
            n197 = property class="Slide (strict)"(reference=w504, "DisabledEnum"=T4."Enabled" ("Disabled")) -> (reference out=w500:refnum<vi>, error out=w499:errorcluster)  [unwired: 1 in]
            n198 = property class="Slide (strict)"(reference=w503, "DisabledEnum"=T4."Enabled" ("Disabled")) -> (reference out=w498:refnum<vi>, error out=w497:errorcluster)  [unwired: 1 in]
            n199 = Close Reference(reference=w502, error in (no error)=w501) -> ()  [unwired: 1 out]
            n200 = Close Reference(reference=w500, error in (no error)=w499) -> ()  [unwired: 1 out]
            n201 = Close Reference(reference=w498, error in (no error)=w497) -> ()  [unwired: 1 out]
          }
          frame True {
            n202 = control-ref of="Pixelclock"() -> (w521:refnum<vi>)
            n203 = control-ref of="Framerate"() -> (w518:refnum<vi>)
            n204 = control-ref of="Exposure"() -> (w516:refnum<vi>)
            n205 = property class="Slide (strict)"(reference=w521, "DisabledEnum"=T4."Disabled and Grayed Out" ("Disabled")) -> (reference out=w514:refnum<vi>, error out=w515:errorcluster)  [unwired: 1 in]
            n206 = property class="Slide (strict)"(reference=w518, "DisabledEnum"=T4."Disabled and Grayed Out" ("Disabled")) -> (reference out=w513:refnum<vi>, error out=w512:errorcluster)  [unwired: 1 in]
            n207 = property class="Slide (strict)"(reference=w516, "DisabledEnum"=T4."Disabled and Grayed Out" ("Disabled")) -> (reference out=w511:refnum<vi>, error out=w510:errorcluster)  [unwired: 1 in]
            n208 = Close Reference(reference=w514, error in (no error)=w515) -> ()  [unwired: 1 out]
            n209 = Close Reference(reference=w513, error in (no error)=w512) -> ()  [unwired: 1 out]
            n210 = Close Reference(reference=w511, error in (no error)=w510) -> ()  [unwired: 1 out]
          }
        }
        n211 = call "uc480_SubVI_Example_MemoryAllocation.vi"(".NET (Reference)"=w446, "Error In"=w443) -> ("Bits/Pixel 2"=→"Bits/Pixel":i32, "Width"=→"Width":i32, "Serial Number"=→"Serial Number":string, "Height"=→"Height":i32, "Error Out"=w483:errorcluster)  [unwired: 13 in]
      }
      frame "Start live" {
        # "Has acquisition started?"
        # "Start Acquisition"
        n212 = property class="Camera"(reference=w547, error in=w548) -> (error out=w557:errorcluster, "Acquisition"=w556:refnum<k24>)  [unwired: 1 out]
        n213 = invoke class="Acquisition" method="HasStarted"(reference=w556, error in=w557) -> (reference out=w552:refnum<k24>, error out=w551:errorcluster, "HasStarted"=w550:i32, "bValue"=w555:bool)  [unwired: 2 in]
        n214 = control-ref of="Load Parameter"() -> (w540:refnum<vi>)
        n215 = control-ref of="Stop Live"() -> (w538:refnum<vi>)
        n216 = control-ref of="Start Live"() -> (w543:refnum<vi>)
        n217 = property class="Bool"(reference=w543, "Disabled"=u8 2 ("Deaktiviert")) -> (reference out=w532:refnum<vi>, error out=w531:errorcluster)  [unwired: 1 in]
        n218 = property class="Bool"(reference=w540, "Disabled"=u8 2 ("Deaktiviert")) -> (reference out=w534:refnum<vi>, error out=w533:errorcluster)  [unwired: 1 in]
        n219 = invoke class="Acquisition" method="ToString"(reference=w552, error in=w551) -> (error out=w554:errorcluster, "ToString"=w553:string)  [unwired: 1 in, 1 out]
        n220 = property class="Bool"(reference=w538, "Disabled"=u8 0 ("Deaktiviert")) -> (reference out=w536:refnum<vi>, error out=w535:errorcluster)  [unwired: 1 in]
        n221 = call "uc480_Error_Handling.vi"("Error Code"=w550, "Error String"=w553, "Error In"=w554) -> ("Error Out"=w549:errorcluster)  [unwired: 8 in]
        n222 = Close Reference(reference=w536, error in (no error)=w535) -> ()  [unwired: 1 out]
        n223 = Close Reference(reference=w532, error in (no error)=w531) -> ()  [unwired: 1 out]
        n224 = Close Reference(reference=w534, error in (no error)=w533) -> ()  [unwired: 1 out]
        n225 = Get Date/Time In Seconds() -> (seconds since 1Jan1904=w526:timestamp)
        n226 = Format Date/Time String(time format string (%c)="%m/%d/%y - %I:%M %p  ", seconds (now)=w526) -> (date/time string=w525:string)  [unwired: 1 in]
        n227 = Concatenate Strings(w525, "Camera started", "\r") -> (w530:string)
        n228 = invoke on="Log" class="Str" method="Append String"("string"=w530) -> (error out=w523:errorcluster)  [unwired: 3 in, 3 out]
        n229 = property on="Log" class="Str"(error in=w523, "Text.Scroll Position"=u32 500000) -> ()  [unwired: 1 in, 2 out]
        n230 = case shown="False" w555 {
          tunnel: [w560 w570] -> w544
          tunnel: w549 -> [w566 w570]
          tunnel: w547 -> [w565 w569]
          tunnel: [w565 w569] -> w546
          frame False {
            w558 = 1 items=["IS_DONT_WAIT", "IS_WAIT"] ("Wait")
            n231 = property class="Camera"(reference=w565, error in=w566) -> (error out=w567:errorcluster, "Acquisition"=w568:refnum<k24>)  [unwired: 1 out]
            n232 = invoke class="Acquisition" method="Capture"(reference=w568, error in=w567, "param"=w558) -> (reference out=w561:refnum<k24>, error out=w562:errorcluster, "Capture"=w559:i32)  [unwired: 1 in, 1 out]
            n233 = invoke class="Acquisition" method="ToString"(reference=w561, error in=w562) -> (error out=w564:errorcluster, "ToString"=w563:string)  [unwired: 1 in, 1 out]
            n234 = call "uc480_Error_Handling.vi"("Error Code"=w559, "Error String"=w563, "Error In"=w564) -> ("Error Out"=w560:errorcluster)  [unwired: 8 in]